vi "attempt-saveImageSeriesHeights.vi"() -> ()   [LabVIEW 2016] (continued)
  out "Match score vs displacement":cluster{dbl[], sgl[]}(graph)={[-2.0, -1.9, -1.8, -1.7, -1.6, -1.5, -1.4, -1.2999999999999998, -1.2, -1.1, -1.0, -0.8999999999999999, -0.7999999999999998, -0.7, -0.5999999999999999, -0.5, -0.3999999999999999, -0.2999999999999998, -0.19999999999999996, -0.09999999999999987, 0.0, 0.10000000000000009, 0.20000000000000018, 0.30000000000000027, 0.40000000000000036, 0.5, 0.6000000000000001, 0.7000000000000002, 0.8000000000000003, 0.9000000000000004, 1.0, 1.1, 1.2000000000000002, 1.3000000000000003, 1.4000000000000004, 1.5, 1.6, 1.7000000000000002, 1.8000000000000003, 1.9000000000000004, 2.0, 2.1000000000000005, 2.2, 2.3, 2.4000000000000004, 2.5, 2.6000000000000005, 2.7, 2.8000000000000007, 2.9000000000000004, 3.0, 3.1000000000000005, 3.2, 3.3000000000000007, 3.4000000000000004, 3.5, 3.6000000000000005, 3.7, 3.8000000000000007, 3.9000000000000004, 4.0, 4.1000000000000005, 4.2, 4.300000000000001, 4.4, 4.5, 4.6000000000000005, 4.7, 4.800000000000001, 4.9, 5.0, 5.1000000000000005, 5.2, 5.300000000000001, 5.4, 5.5, 5.6000000000000005, 5.7, 5.800000000000001, 5.9, 6.0, 6.1, 6.200000000000001, 6.300000000000001, 6.4, 6.5, 6.6, 6.700000000000001, 6.800000000000001, 6.9, 7.0, 7.1, 7.200000000000001, 7.300000000000001, 7.4, 7.5, 7.600000000000001, 7.700000000000001, 7.800000000000001, 7.9, 8.0], [879.0314, 880.5322, 881.50525, 883.59375, 885.04114, 886.6321, 887.99164, 889.89014, 891.54895, 892.7096, 894.01355, 895.76086, 896.38574, 897.8513, 899.14215, 900.46564, 901.9159, 903.5967, 905.61066, 907.6271, 909.8519, 911.7539, 914.30066, 916.9432, 919.2109, 922.02893, 925.1449, 927.1994, 930.3543, 933.7616, 937.412, 941.27527, 945.56866, 949.7169, 954.40594, 958.87146, 964.12915, 966.3607, 971.17303, 975.7742, 979.7761, 983.59674, 986.48694, 988.4218, 989.78876, 991.7045, 990.82227, 992.4532, 993.7908, 994.56085, 994.9838, 995.4237, 995.7052, 996.1429, 996.40594, 995.1158, 994.9518, 994.49426, 993.5686, 991.30493, 988.9285, 985.62024, 979.23346, 976.25146, 972.1395, 967.325, 962.50824, 957.11816, 951.9495, 947.2621, 943.3269, 939.42737, 936.4822, 934.05096, 931.73193, 929.0479, 926.9251, 923.81866, 921.44275, 919.72864, 917.4266, 914.7757, 913.0611, 911.3056, 910.391, 910.2793, 909.92053, 909.1891, 908.61414, 907.92114, 906.2847, 905.24835, 904.1167, 902.81866, 901.4715, 900.2599, 898.7702, 897.3308, 896.09454, 894.80115, 893.3429]}
  in  "Match position variation tolerance":sgl=0.25
  out "Z step":dbl=10.0
  out "Image":T1(plugin-control)
  in  "End Z [mm]":dbl=8.0
  in  "Stepsize [mm]":dbl=0.1
  out "Matches (pixel)":T2(array[cluster])=[{"Position"={"x"=1127.198, "y"=915.98065}, "Angle"=0.0, "Scale"=1.0, "Score"=893.3429, "Bounding Box"=[{"x"=974.198, "y"=763.98065}, {"x"=1280.198, "y"=763.98065}, {"x"=1280.198, "y"=1067.9807}, {"x"=974.198, "y"=1067.9807}, {"x"=974.198, "y"=763.98065}]}, {"Position"={"x"=1514.1495, "y"=359.13376}, "Angle"=0.0, "Scale"=1.0, "Score"=588.01715, "Bounding Box"=[{"x"=1361.1495, "y"=207.13376}, {"x"=1667.1495, "y"=207.13376}, {"x"=1667.1495, "y"=511.13376}, {"x"=1361.1495, "y"=511.13376}, {"x"=1361.1495, "y"=207.13376}]}, {"Position"={"x"=530.31506, "y"=1381.0135}, "Angle"=0.0, "Scale"=1.0, "Score"=572.6888, "Bounding Box"=[{"x"=377.31506, "y"=1229.0135}, {"x"=683.31506, "y"=1229.0135}, {"x"=683.31506, "y"=1533.0135}, {"x"=377.31506, "y"=1533.0135}, {"x"=377.31506, "y"=1229.0135}]}, {"Position"={"x"=1194.1893, "y"=1528.8197}, "Angle"=0.0, "Scale"=1.0, "Score"=556.0711, "Bounding Box"=[{"x"=1041.1893, "y"=1376.8197}, {"x"=1347.1893, "y"=1376.8197}, {"x"=1347.1893, "y"=1680.8197}, {"x"=1041.1893, "y"=1680.8197}, {"x"=1041.1893, "y"=1376.8197}]}, {"Position"={"x"=129.51509, "y"=1364.8577}, "Angle"=0.0, "Scale"=1.0, "Score"=534.0569, "Bounding Box"=[{"x"=-23.48491, "y"=1212.8577}, {"x"=282.51508, "y"=1212.8577}, {"x"=282.51508, "y"=1516.8577}, {"x"=-23.48491, "y"=1516.8577}, {"x"=-23.48491, "y"=1212.8577}]}, {"Position"={"x"=1668.3909, "y"=1350.8374}, "Angle"=0.0, "Scale"=1.0, "Score"=523.21924, "Bounding Box"=[{"x"=1515.3909, "y"=1198.8374}, {"x"=1821.3909, "y"=1198.8374}, {"x"=1821.3909, "y"=1502.8374}, {"x"=1515.3909, "y"=1502.8374}, {"x"=1515.3909, "y"=1198.8374}]}, {"Position"={"x"=120.40187, "y"=1854.9404}, "Angle"=0.0, "Scale"=1.0, "Score"=515.30743, "Bounding Box"=[{"x"=-32.59813, "y"=1702.9404}, {"x"=273.40186, "y"=1702.9404}, {"x"=273.40186, "y"=2006.9404}, {"x"=-32.59813, "y"=2006.9404}, {"x"=-32.59813, "y"=1702.9404}]}, {"Position"={"x"=840.2334, "y"=1425.0645}, "Angle"=0.0, "Scale"=1.0, "Score"=508.74185, "Bounding Box"=[{"x"=687.2334, "y"=1273.0645}, {"x"=993.2334, "y"=1273.0645}, {"x"=993.2334, "y"=1577.0645}, {"x"=687.2334, "y"=1577.0645}, {"x"=687.2334, "y"=1273.0645}]}, {"Position"={"x"=1681.2684, "y"=805.9706}, "Angle"=0.0, "Scale"=1.0, "Score"=501.45316, "Bounding Box"=[{"x"=1528.2684, "y"=653.9706}, {"x"=1834.2684, "y"=653.9706}, {"x"=1834.2684, "y"=957.9706}, {"x"=1528.2684, "y"=957.9706}, {"x"=1528.2684, "y"=653.9706}]}] {"Bounding Box"."y" format="%.2f"; "Bounding Box"."x" format="%.2f"; "Score" format="%.2f"; "Scale" format="%.2f"; "Angle" format="%.2f"; "Position"."y" format="%.2f"; "Position"."x" format="%.2f"}
  in  "Match parameters":T3={"Number of Matches Requested"=10, "Minimum Match Score"=500.0, "Angle Ranges"=[]}
  in  "Template File Path":path=path "E:/XYZstage+Camera_CollectedImages/12-14-2016/test_sub_smallerDot_-685,-128,3p4.png"
  in  "Axes Speeds [mm/s]":T4={"X Speed"=25.0, "Y Speed"=5.0, "Z Speed"=1.0}
  in  "Initial Location [mm]":T5={"Go to X"=-685.0, "Go to Y"=-128.0, "Go to Z"=-2.0}
  out "Intensity histogram":T6(graph)={"Starting Value"=0.0, "Incremental Value"=1.0, "Histogram"=[0, 150, 32506, 224440, 72176, 32514, 24980, 20375, 14194, 28017, 104301, 253038, 323157, 301095, 227717, 209323, 173693, 175646, 161707, 128964, 105278, 82020, 84233, 81813, 93253, 96135, 110312, 107820, 127805, 130789, 152441, 156182, 178245, 162226, 149895, 115876, 98993, 74348, 64510, 51354, 47133, 38158, 37497, 33782, 33023, 26163, 21842, 15148, 11810, 8588, 7813, 6201, 4673, 4086, 3220, 2494, 1799, 1446, 1003, 718, 376, 228, 88, 29, 7, 2, 0, 0, 0, 0, 0, 0, 0, 0, 0, 0, 0, 0, 0, 0, 0, 0, 0, 0, 0, 0, 0, 0, 0, 0, 0, 0, 0, 0, 0, 0, 0, 0, 0, 0, 0, 0, 0, 0, 0, 0, 0, 0, 0, 0, 0, 0, 0, 0, 0, 0, 0, 0, 0, 0, 0, 0, 0, 0, 0, 0, 0, 0, 0, 0, 0, 0, 0, 0, 0, 0, 0, 0, 0, 0, 0, 0, 0, 0, 0, 0, 0, 0, 0, 0, 0, 0, 0, 0, 0, 0, 0, 0, 0, 0, 0, 0, 0, 0, 0, 0, 0, 0, 0, 0, 0, 0, 0, 0, 0, 0, 0, 0, 0, 0, 0, 0, 0, 0, 0, 0, 0, 0, 0, 0, 0, 0, 0, 0, 0, 0, 0, 0, 0, 0, 0, 0, 0, 0, 0, 0, 0, 0, 0, 0, 0, 0, 0, 0, 0, 0, 0, 0, 0, 0, 0, 0, 0, 0, 0, 0, 0, 0, 0, 0, 0, 0, 0, 0, 0, 0, 0, 0, 0, 0, 0, 0, 0, 0, 0, 0, 0, 0, 0, 0, 0, 0, 0, 0, 0, 0]}
  out "Moving":bool
  out "XYZ Stage Current Position":T7={"X [-750, 750 mm]"=-684.9998825073242, "Y [-150, 30 mm]"=-128.00212852478026, "Z [-50, 50 mm]"=7.9998000000000005}
  out "Error report":errorcluster
  in  "Camera Name":refnum<k21>="cam0" caption="IMAQdx Session"
  # "ANALYSIS"
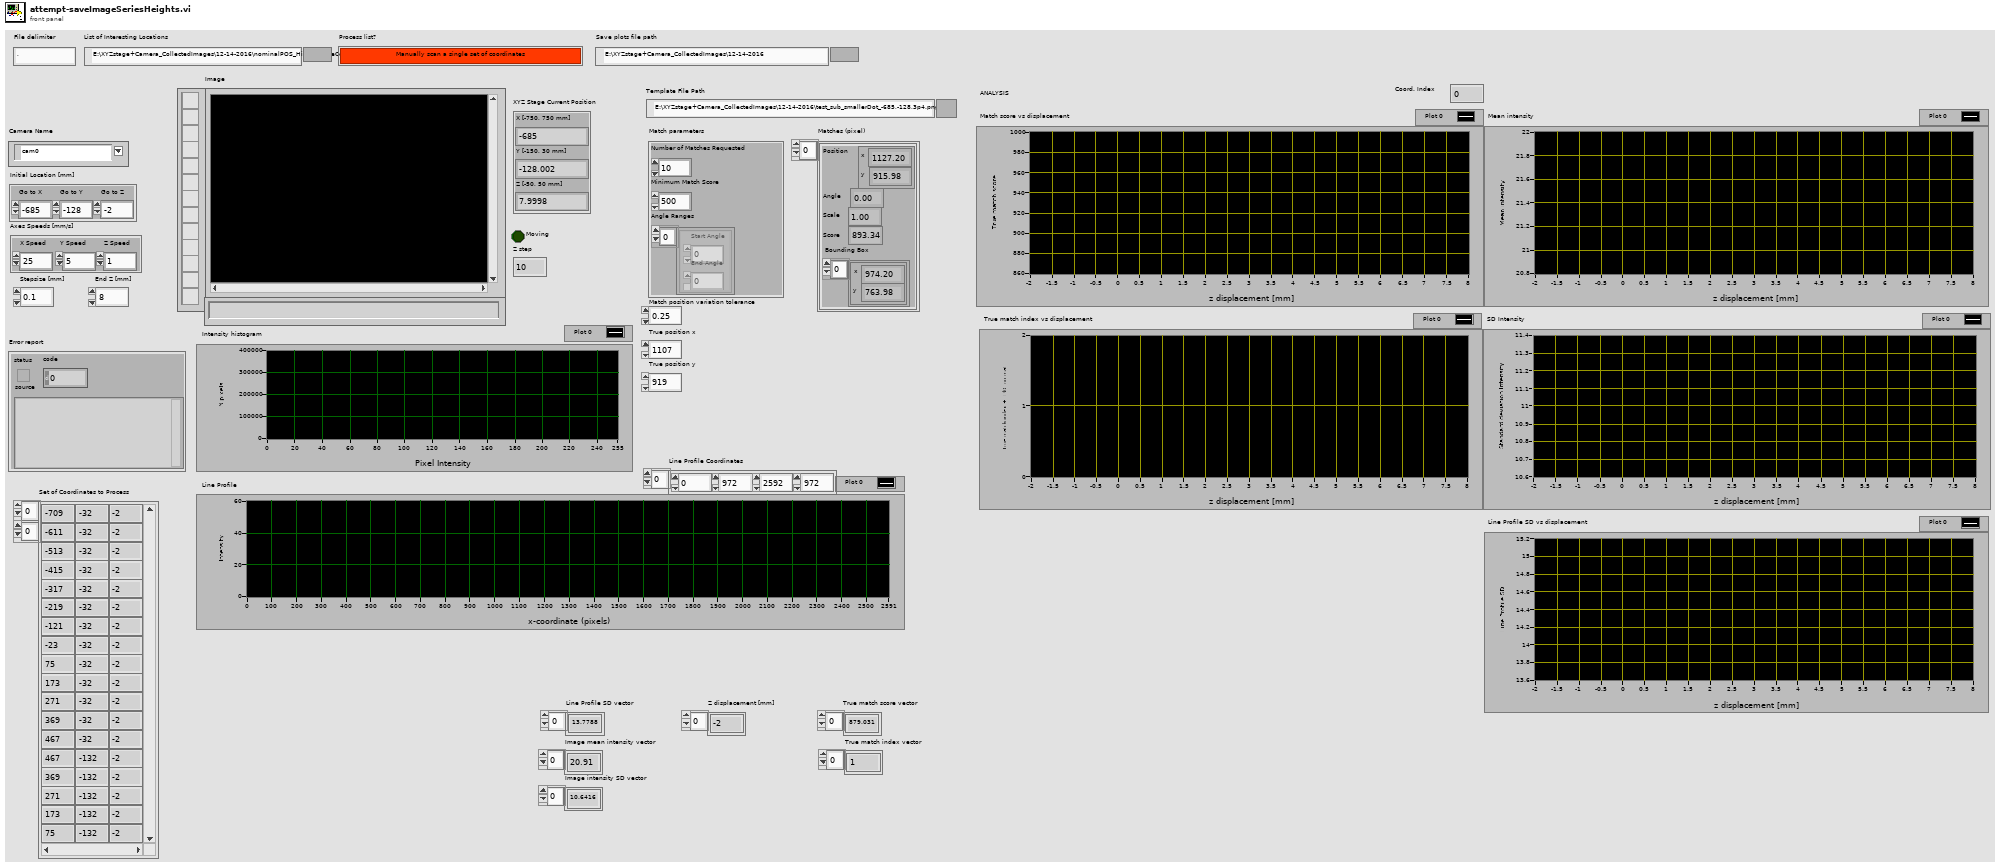
[diagram p1: front panel]
types:
  T1 = typedef "IMAQ Image.ctl" = refnum<image>
  T2 = cluster{"Position":cluster{"x":sgl, "y":sgl}, "Angle":sgl, "Scale":sgl, "Score":sgl, "Bounding Box":cluster{"x":sgl, "y":sgl}[]}[]
  T3 = cluster{"Number of Matches Requested":i32, "Minimum Match Score":sgl, "Angle Ranges":cluster{"Start Angle":sgl, "End Angle":sgl}[]}
  T4 = cluster{"X Speed":dbl, "Y Speed":dbl, "Z Speed":dbl}
  T5 = cluster{"Go to X":dbl, "Go to Y":dbl, "Go to Z":dbl}
  T6 = cluster{"Starting Value":sgl, "Incremental Value":sgl, "Histogram":u32[]}
  T7 = cluster{"X [-750, 750 mm]":dbl, "Y [-150, 30 mm]":dbl, "Z [-50, 50 mm]":dbl}
  T8 = cluster{"Set of Coordinates to Process[0]":dbl, "Set of Coordinates to Process[1]":dbl, "Set of Coordinates to Process[2]":dbl}
  T9 = typedef "Image Type" = u32
  T10 = typedef "IMAQdx.ctl" = refnum<k21>
  T11 = cluster{"Final X":dbl, "Final Y":dbl, "Final Z":dbl}
  T12 = cluster{"Min":sgl, "Max":sgl, "Mean":sgl, "Std Dev":sgl, "Count":i32}
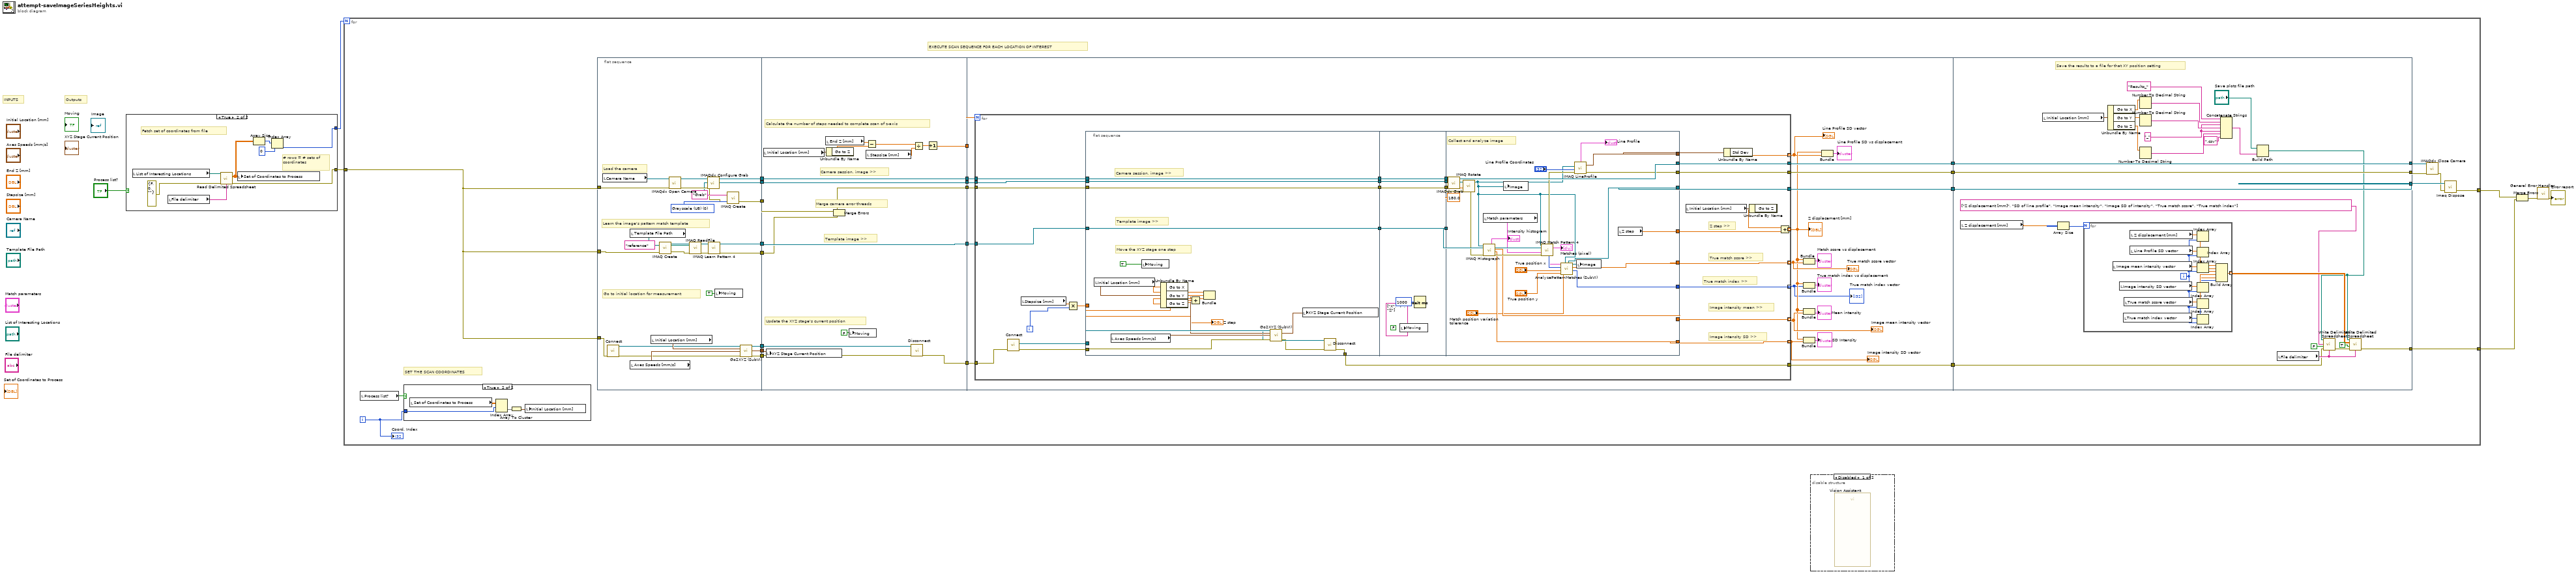
[diagram p0: block diagram]
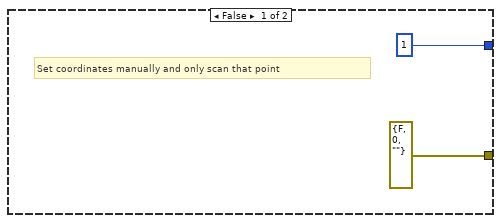
[diagram p2: hidden frame]
diagram:
  # "Outputs"
  # "INPUTS"
  n1 = case shown="True" "Process list?" {
    tunnel: [1 w12] -> w2
    tunnel: [errorcluster {"status"=FALSE, "code"=0, "source"=""} ("error in (no error)") w10] -> w3
    frame False {
      # "Set coordinates manually and only scan that point"
    }
    frame True {
      # "# rows = # sets of\ncoordinates"
      # "Fetch set of coordinates from file"
      n2 = local read "List of Interesting Locations"() -> (w16:path)
      n3 = local read "File delimiter"() -> (w17:string)
      n4 = call-poly <vilib>:"Read Delimited Spreadsheet.vi"("file path (dialog if empty)"=w16, "error in (no error)"=errorcluster {"status"=FALSE, "code"=0, "source"=""}, "delimiter (\\t)"=w17) -> ("all rows"=w15:dbl[][], "error out"=w10:errorcluster)  [unwired: 7 in, 4 out]
      n5 = local write "Set of Coordinates to Process"(w15) -> ()
      n6 = Array Size(array=w15) -> (size(s)=w14:i32[])
      n7 = Index Array(array=w14, index=0) -> (element=w12:i32)
    }
  }
  n8 = for {
    N: w2 -> [_]
    tunnel: [w30] -> w6
    tunnel: w3 -> [w18]
    tunnel: [w19] -> w1
    i -> [w27]
    # "SET THE SCAN COORDINATES"
    # "EXECUTE SCAN SEQUENCE FOR EACH LOCATION OF INTEREST"
    n9 = local read "Process list?"() -> (w28:bool)
    n10 = case shown="True" w28 {
      tunnel: w27 -> [_ w47]
      frame False {
      }
      frame True {
        n11 = local read "Set of Coordinates to Process"() -> (w48:dbl[][])
        n12 = Index Array(array=w48, index (row)=w47) -> (element=w46:dbl[])  [unwired: 1 in]
        n13 = Array To Cluster(array=w46) -> (cluster=w45:T8)
        n14 = local write "Initial Location [mm]"(w45) -> ()
      }
    }
    n15 = flat-sequence {
      tunnel: [w76] -> w44
      tunnel: [w75] -> w43
      tunnel: [w70] -> w42
      tunnel: [w59] -> w41
      tunnel: [w55] -> w40
      tunnel: [w54] -> w39
      tunnel: [w53] -> w38
      tunnel: [w52] -> w37
      tunnel: w18 -> [w51]
      tunnel: w18 -> [w50]
      tunnel: w18 -> [w49]
      tunnel: w44 -> [w89]
      tunnel: w43 -> [w88]
      tunnel: w42 -> [w93]
      tunnel: [w77] -> w36
      tunnel: [w87] -> w35
      tunnel: [w85] -> w34
      tunnel: w41 -> [w85]
      tunnel: w40 -> [w84]
      tunnel: [w84] -> w33
      tunnel: w39 -> [w82]
      tunnel: [w80] -> w32
      tunnel: [w83] -> w31
      tunnel: w38 -> [w83]
      tunnel: w37 -> [w81]
      tunnel: w36 -> [w107]
      tunnel: w35 -> [w115]
      tunnel: w34 -> [w114]
      tunnel: w33 -> [w113]
      tunnel: w32 -> [w112]
      tunnel: w31 -> [w111]
      tunnel: [w110] -> w26
      tunnel: [w109] -> w25
      tunnel: [w108] -> w24
      tunnel: [w102] -> w23
      tunnel: [w227] -> w21
      tunnel: [w228] -> w22
      tunnel: [w207] -> w29
      tunnel: w26 -> [w207]
      tunnel: w25 -> [w204]
      tunnel: w24 -> [w228]
      tunnel: w23 -> [w227]
      tunnel: [w203] -> w19
      frame #0 {
        w57 = T9 0 items=["Grayscale (U8)", "Grayscale (I16)", "Grayscale (SGL)", "Complex (CSG)", "RGB (U32)", "HSL (U32)", "RGB (U64)", "Grayscale (U16)"] ("Image Type")
        # "Learn the image's pattern match template"
        # "Load the camera"
        # "Go to initial location for measurement"
        n16 = local read "Camera Name"() -> (w68:refnum<k21>)
        n17 = call "Connect.vi"("error in (no error)"=w49) -> ("error out"=w69:errorcluster, "controller"=w71:refnum<k24>)  [unwired: 9 in]
        n18 = local read "Template File Path"() -> (w65:path)
        n19 = local read "Axes Speeds [mm/s]"() -> (w73:T4)
        n20 = local read "Initial Location [mm]"() -> (w72:T5)
        n21 = call "IMAQ Create"("Image Name"="reference", "error in (no error)"=w51) -> ("New Image"=w64:T1, "error out"=w63:errorcluster)  [unwired: 3 in]
        n22 = call <vilib>:"IMAQdx Open Camera.vi"("error in"=w50, "Session In"=w68) -> ("error out"=w66:errorcluster, "Session Out"=w67:T10)  [unwired: 1 in, 7 out]
        n23 = call "IMAQ ReadFile"("File Path"=w65, "error in (no error)"=w63, "Image"=w64) -> ("error out"=w60:errorcluster, "Image Out"=w61:T1)  [unwired: 4 in, 3 out]
        n24 = call <vilib>:"IMAQdx Configure Grab.vi"("error in"=w66, "Session In"=w67) -> ("error out"=w56:errorcluster, "Session Out"=w59:T10)  [unwired: 8 out]
        n25 = call "IMAQ Learn Pattern 4"("error in (no error)"=w60, "Image"=w61) -> ("error out"=w52:errorcluster, "Template Image Out"=w53:T1)  [unwired: 7 in, 1 out]
        n26 = local write "Moving"(TRUE ("Moving")) -> ()
        n27 = call "IMAQ Create"("Image Name"="Grab", "Image Type"=w57, "error in (no error)"=w56) -> ("New Image"=w55:T1, "error out"=w54:errorcluster)  [unwired: 1 in, 1 out]
        n28 = call "Go2XYZ (SubVI).vi"(".NET Refnum in"=w71, "Go to Coordinates"=w72, "Axis Speeds"=w73, "error in (no error)"=w69) -> (".NET Refnum out"=w76:refnum<k24>, "Final Position"=w70:T11, "error out"=w75:errorcluster)  [unwired: 8 in, 1 out]
      }
      frame #1 {
        # "Merge camera error threads"
        # "Camera session, image >>"
        # "Template image >>"
        # "Calculate the number of steps needed to complete scan of z-axis"
        # "Update the XYZ stage's current position"
        n29 = local read "Initial Location [mm]"() -> (w92:T5)
        n30 = local write "XYZ Stage Current Position"(w93) -> ()
        n31 = local read "End Z [mm]"() -> (w79:dbl)
        n32 = Unbundle By Name(w92) -> ("Go to Z"=w91:dbl)
        n33 = Merge Errors(w82, w81) -> (w80:errorcluster)
        n34 = local write "Moving"(FALSE ("Moving")) -> ()
        n35 = Subtract(x=w79, y=w91) -> (x-y=w90:dbl)
        n36 = local read "Stepsize [mm]"() -> (w86:dbl)
        n37 = call "Disconnect.vi"("error in (no error)"=w88, "controller"=w89) -> ("error out"=w87:errorcluster)  [unwired: 9 in]
        n38 = Divide(x=w90, y=w86) -> (x/y=w78:dbl)
        n39 = Increment(x=w78) -> (x+1=w77:dbl)
      }
      frame #2 {
        n40 = for {
          N: w107 -> [_]
          tunnel: w115 -> [w144]
          tunnel: w114 -> [w142]
          tunnel: w113 -> [w141]
          tunnel: w112 -> [w140]
          tunnel: w111 -> [w139]
          tunnel: [w138] -> w110
          tunnel: [w137] -> w109
          tunnel: [w136] -> w108
          tunnel: [w130] -> w98 mode=indexing
          tunnel: [w135] -> w106 mode=indexing
          tunnel: [w134] -> w105 mode=indexing
          tunnel: [w133] -> w104 mode=indexing
          tunnel: [w132] -> w102
          tunnel: [w119] -> w96 mode=indexing
          tunnel: [w116] -> w95 mode=indexing
          i -> [w146]
          (unwired) string[] ["X", "Y", "Z"] ("Axes Names")
          # "True match index >>"
          # "Image intensity SD >>"
          # "Image intensity mean >>"
          # "True match score >>"
          # "Z step >>"
          n41 = call "Connect.vi"("error in (no error)"=w144) -> ("error out"=w118:errorcluster, "controller"=w147:refnum<k24>)  [unwired: 9 in]
          n42 = local read "Stepsize [mm]"() -> (w143:dbl)
          n43 = Multiply(x=w143, y=w146) -> (x*y=w145:dbl)
          n44 = flat-sequence {
            tunnel: w147 -> [w166]
            tunnel: w118 -> [w165]
            tunnel: w145 -> [w148]
            tunnel: [w153] -> w127
            tunnel: w142 -> [w153]
            tunnel: w141 -> [w152]
            tunnel: [w152] -> w125
            tunnel: w140 -> [w151]
            tunnel: [w151] -> w123
            tunnel: [w150] -> w121
            tunnel: w139 -> [w150]
            tunnel: [w149] -> w137
            tunnel: w127 -> [w172]
            tunnel: [w172] -> w126
            tunnel: w125 -> [w171]
            tunnel: [w171] -> w124
            tunnel: w123 -> [w170]
            tunnel: [w170] -> w122
            tunnel: w121 -> [w169]
            tunnel: [w169] -> w120
            tunnel: w126 -> [w202]
            tunnel: w124 -> [w201]
            tunnel: w122 -> [w200]
            tunnel: w120 -> [w198]
            tunnel: [w191] -> w138
            tunnel: [w196] -> w136
            tunnel: [w194] -> w128
            tunnel: [w184] -> w135
            tunnel: [w193] -> w134
            tunnel: [w192] -> w133
            tunnel: [w180] -> w132
            tunnel: [w183] -> w119
            tunnel: [w178] -> w117
            frame #0 {
              # "Camera session, image >>"
              # "Template image >>"
              # "Move the XYZ stage one step"
              n45 = local read "Initial Location [mm]"() -> (w162:T5)
              n46 = local read "Axes Speeds [mm/s]"() -> (w163:T4)
              n47 = local write "Moving"(TRUE ("Moving")) -> ()
              n48 = Unbundle By Name(w162) -> ("Go to X"=w158:dbl, "Go to Y"=w159:dbl, "Go to Z"=w161:dbl)
              n49 = Add(x=w161, y=w148) -> (x+y=w160:dbl)
              n50 = Bundle("Go to X"=w158, "Go to Y"=w159, w160) -> (w157:cluster{"Go to X":dbl, "Go to Y":dbl, dbl})  [unwired: 1 in]
              n51 = call "Go2XYZ (SubVI).vi"(".NET Refnum in"=w166, "Go to Coordinates"=w157, "Axis Speeds"=w163, "error in (no error)"=w165) -> (".NET Refnum out"=w156:refnum<k24>, "Final Position"=w154:T11, "error out"=w155:errorcluster)  [unwired: 8 in, 1 out]
              n52 = local write "XYZ Stage Current Position"(w154) -> ()
              n53 = call "Disconnect.vi"("error in (no error)"=w155, "controller"=w156) -> ("error out"=w149:errorcluster)  [unwired: 9 in]
              "Z step" <- w148
            }
            frame #1 {
              n54 = local write "Moving"(FALSE ("Moving")) -> ()
              n55 = Wait (ms)(milliseconds to wait=u32 1000) -> ()  [unwired: 1 out]
            }
            frame #2 {
              # "Collect and analyze image"
              n56 = call <vilib>:"IMAQdx Grab.vi"("error in"=w200, "Image In"=w201, "Session In"=w202) -> ("error out"=w176:errorcluster, "Image Out"=w177:T1, "Session Out"=w196:T10)  [unwired: 1 in, 5 out]
              n57 = call "IMAQ Rotate"("error in (no error)"=w176, "Angle (degrees)"=sgl 180.0, "Image Src"=w177) -> ("error out"=w175:errorcluster, "Image Dst Out"=w173:T1)  [unwired: 7 in]
              n58 = local read "Match parameters"() -> (w197:T3)
              n59 = call "IMAQ Histograph"("error in (no error)"=w175, "Image"=w173) -> ("error out"=w199:errorcluster, "Standard  Deviation"=w192:sgl, "Mean Value"=w193:sgl, "Histogram Graph"=→"Intensity histogram":T6)  [unwired: 6 in]
              n60 = local write "Image"(w173) -> ()
              n61 = call "IMAQ Match Pattern 4"("Image"=w173, "Template Image"=w198, "Parameters"=w197, "error in (no error)"=w199) -> ("Matches (pixel)"=w188:T2, "Number of Matches"=w189:i32, "error out"=w179:errorcluster)  [unwired: 7 in, 2 out]
              "Matches (pixel)" <- w188
              n62 = call "AnalyzePatternMatches (SubVI).vi"("Match position variation tolerance"="Match position variation tolerance", "Image in"=w173, "true y"="True position y", "true x"="True position x", "Number of Matches"=w189, "Matches (pixel)"=w188) -> ("True Match Index"=w183:i32, "True Match Score"=w184:sgl, "Display with box"=w190:T1, "Image out"=w191:T1)  [unwired: 2 in]
              n63 = call "IMAQ LineProfile"("error in (no error)"=w179, "Line Coordinates"="Line Profile Coordinates", "Image"=w173) -> ("error out"=w180:errorcluster, "Line Graph"=→"Line Profile":cluster{"x0":sgl, "dx":sgl, "Pixels Line":sgl[]}, "Line Information"=w178:T12)  [unwired: 2 in, 1 out]
              n64 = local write "Image"(w190) -> ()
              n65 = local read "Z step"() -> (w194:dbl)
            }
          }
          n66 = local read "Initial Location [mm]"() -> (w131:T5)
          n67 = Unbundle By Name(w117) -> ("Std Dev"=w116:sgl)
          n68 = Unbundle By Name(w131) -> ("Go to Z"=w129:dbl)
          n69 = Add(x=w129, y=w128) -> (x+y=w130:dbl)
        }
        "Line Profile SD vector" <- w95
        "Z displacement [mm]" <- w98
        "Image mean intensity vector" <- w105
        "Image intensity SD vector" <- w104
        "True match score vector" <- w106
        "True match index vector" <- w96
        n70 = Bundle(w98, w106) -> (→"Match score vs displacement":cluster{dbl[], sgl[]})  [unwired: 1 in]
        n71 = Bundle(w98, w96) -> (→"True match index vs displacement":cluster{dbl[], i32[]})  [unwired: 1 in]
        n72 = Bundle(w98, w105) -> (→"Mean intensity":cluster{dbl[], sgl[]})  [unwired: 1 in]
        n73 = Bundle(w98, w104) -> (→"SD Intensity":cluster{dbl[], sgl[]})  [unwired: 1 in]
        n74 = Bundle(w98, w95) -> (→"Line Profile SD vs displacement":cluster{dbl[], sgl[]})  [unwired: 1 in]
      }
      frame #3 {
        w215 = "_"
        # "Save the results to a file for that XY position setting"
        n75 = local read "Z displacement [mm]"() -> (w220:dbl[])
        n76 = local read "Initial Location [mm]"() -> (w209:T5)
        n77 = Array Size(array=w220) -> (size(s)=w221:i32)
        n78 = for {
          N: w221 -> [_]
          tunnel: [w240] -> w225 mode=indexing
          i -> [w232]
          n79 = local read "Image mean intensity vector"() -> (w238:sgl[])
          n80 = local read "Image intensity SD vector"() -> (w237:sgl[])
          n81 = local read "True match index vector"() -> (w233:i32[])
          n82 = local read "True match score vector"() -> (w231:sgl[])
          n83 = local read "Z displacement [mm]"() -> (w242:dbl[])
          n84 = local read "Line Profile SD vector"() -> (w239:sgl[])
          n85 = Index Array(array=w242, index=w232) -> (element=w241:dbl)
          n86 = Index Array(array=w239, index=w232) -> (element=w236:sgl)
          n87 = Index Array(array=w238, index=w232) -> (element=w235:sgl)
          n88 = Index Array(array=w237, index=w232) -> (element=w234:sgl)
          n89 = Index Array(array=w231, index=w232) -> (element=w230:sgl)
          n90 = Index Array(array=w233, index=w232) -> (element=w229:i32)
          n91 = Build Array(w241, w236, w235, w234, w230, w229) -> (w240:dbl[])
        }
        n92 = Unbundle By Name(w209) -> ("Go to X"=w210:dbl, "Go to Y"=w211:dbl, "Go to Z"=w212:dbl)
        n93 = Number To Decimal String(number=w210) -> (decimal integer string=w214:string)  [unwired: 1 in]
        n94 = Number To Decimal String(number=w211) -> (decimal integer string=w216:string)  [unwired: 1 in]
        n95 = Number To Decimal String(number=w212) -> (decimal integer string=w217:string)  [unwired: 1 in]
        n96 = Concatenate Strings("Results_", w214, w215, w216, w215, w217, ".csv" ("string")) -> (w219:string)
        n97 = Build Path(base path="Save plots file path", name or relative path=w219) -> (appended path=w205:path)
        n98 = local read "File delimiter"() -> (w226:string)
        n99 = call-poly <vilib>:"Write Delimited Spreadsheet.vi"("file path (dialog if empty)"=w205, "1D data"=string[] ["Z displacement [mm]", "SD of line profile", "Image mean intensity", "Image SD of intensity", "True match score", "True match index"], "append to file? (new file:F)"=FALSE, "error in (no error)"=w204, "delimiter (\\t)"=w226) -> ("error out"=w224:errorcluster)  [unwired: 9 in, 1 out]
        n100 = call-poly <vilib>:"Write Delimited Spreadsheet.vi"("file path (dialog if empty)"=w205, "2D data"=w225, "append to file? (new file:F)"=TRUE, "error in (no error)"=w224, "delimiter (\\t)"=w226) -> ("error out"=w203:errorcluster)  [unwired: 9 in, 1 out]
      }
    }
    n101 = call <vilib>:"IMAQdx Close Camera.vi"("error in"=w21, "Session In"=w22) -> ("error out"=w20:errorcluster)  [unwired: 9 out]
    n102 = call "Imaq Dispose"("Image"=w29, "error in (no error)"=w20) -> ("error out"=w30:errorcluster)  [unwired: 4 in]
    "Coord. Index" <- w27
  }
  n103 = disable-structure shown="Disabled" {
    frame Disabled {
      n104 = call "Vision Assistant"() -> ()  [unwired: 25 in, 3 out]
    }
    frame Enabled {
    }
  }
  n105 = Merge Errors(w6, w1) -> (w5:errorcluster)
  n106 = call <vilib>:"General Error Handler.vi"("error in (no error)"=w5) -> ("error out"=→"Error report":errorcluster)  [unwired: 2 in, 12 out]
